vi "UHR-Fleezers Control (host) - Avogadro v1.vi"() -> ()   [LabVIEW 2014] (continued)
            n459 = local write "Stage Moving"(TRUE ("Stage Moving")) -> ()
            n460 = local write "Start Saving"(TRUE ("Start Saving")) -> ()
            n461 = call "Set Stage Position.vi"("Position"=w813, "error in"=w812, "VISA resource name in"=w811) -> ("error out"=w809:errorcluster, "VISA resource name out"=w810:refnum<visa-resource-name>)  [unwired: 1 out]
          }
          frame #2 {
            # "go back to start"
            n462 = call "Set Stage Position.vi"("Position"=w815, "error in"=w816, "VISA resource name in"=w817) -> ()  [unwired: 3 out]
          }
          frame #3 {
            # "stop saving"
            n463 = local write "Stop Saving"(TRUE ("Stop Saving")) -> ()
            n464 = local write "Stage Moving"(FALSE ("Stage Moving")) -> ()
          }
        }
      }
      event "Move to Position 1", "Move to Position 2", "Move to Position 3", "Move to Position 4", "Move to Position 5", "Lower Ch. Cap.", "Move to Position 6": Value Change {
        w820 = FALSE
        n465 = event-data() -> ()  [unwired: 1 in, 5 out]
        n466 = Or(x="Move to Position 5", y="Lower Ch. Cap.") -> (x .or. y?=w825:bool)
        n467 = Build Array("Move to Position 1", "Move to Position 2", "Move to Position 3", "Move to Position 4", w825, "Move to Position 6") -> (w828:bool[])
        n468 = local write "Move to Position 1"(w820) -> ()
        n469 = local write "Move to Position 2"(w820) -> ()
        n470 = local write "Move to Position 3"(w820) -> ()
        n471 = local write "Move to Position 4"(w820) -> ()
        n472 = local write "Move to Position 5"(w820) -> ()
        n473 = local write "Move to Position 6"(w820) -> ()
        n474 = Boolean Array To Number(Boolean array=w828) -> (number=w827:u32)
        n475 = Logarithm Base 2(1:w827) -> (0:w826:dbl)
        n476 = flat-sequence {
          tunnel: w826 -> [w837]
          tunnel: w823 -> [w835]
          tunnel: w822 -> [w834]
          frame #0 {
            n477 = local read "Saved Stage Positions"() -> (w845:dbl[][])
            n478 = Array Subset(array=w845, index (row)=w837, length (row)=1 ("length"), index (col)=1 ("index"), length (col)=3 ("length")) -> (w842:dbl[][])
            n479 = Reshape Array(w842, 3 ("dimension size")) -> (w840:dbl[])
            n480 = Array To Cluster(array=w840) -> (cluster=w839:cluster{"[0]":dbl, "[1]":dbl, "[2]":dbl})
            n481 = call "Set Stage Position.vi"("Position"=w839, "error in"=w834, "VISA resource name in"=w835) -> ("error out"=w838:errorcluster)  [unwired: 2 out]
            n482 = local write "Stage Moving"(TRUE ("Stage Moving")) -> ()
            n483 = local write "Stage Control Serial Error"(w838) -> ()
          }
          frame #1 {
            n484 = local write "Stage Moving"(FALSE ("Stage Moving")) -> ()
            n485 = call <vilib>:"Beep.vi"() -> ()  [unwired: 3 in, 9 out]
          }
        }
      }
      event "Force FB Data\nScript": Value Change {
        n486 = event-data() -> ()  [unwired: 1 in, 5 out]
        n487 = flat-sequence {
          tunnel: w853 -> [w857]
          tunnel: w854 -> [w858]
          tunnel: [w858] -> w849
          tunnel: [w857] -> w848
          tunnel: w849 -> [w861]
          tunnel: w848 -> [w860]
          tunnel: ["Trap Trig Fl."] -> w850
          tunnel: [w886] -> w851
          tunnel: w850 -> [w886]
          tunnel: [w890] -> w852
          tunnel: w851 -> [w890]
          tunnel: w852 -> [w892]
          frame #0 {
            n488 = property on="Trap Delta (MHz)" class="DigNum (strict)"("Val(Sgnl)"="Trap Delta Before Moving") -> ()  [unwired: 2 in, 2 out]
          }
          frame #1 {
            n489 = local read "Saved Stage Positions"() -> (w863:dbl[][])
            n490 = property on="Trap Pos. FB Offset Factor" class="DigNum (strict)"("Val(Sgnl)"=i64 0 ("Value (Signaling)")) -> ()  [unwired: 2 in, 2 out]
            n491 = local write "FB Trap Pos Offset"(0.0 ("FB Trap Pos Offset")) -> ()
            n492 = local write "Stage Moving"(TRUE ("Stage Moving")) -> ()
            n493 = call "move to saved stage position.vi"("error in"=w860, "Stage VISA resource name in"=w861, "Position"="Stage Position To Establish FB", "Saved Stage Positions"=w863) -> ("error out"=w859:errorcluster)  [unwired: 1 out]
            n494 = local write "Stage Control Serial Error"(w859) -> ()
          }
          frame #2 {
            n495 = call <vilib>:"Beep.vi"() -> ()  [unwired: 3 in, 9 out]
            n496 = Multiply(x="Wait (s)", y=u32 1000 ("milliseconds to wait")) -> (x*y=w870:u32)
            n497 = property on="Trap Delta (MHz)" class="DigNum (strict)"("Val(Sgnl)"="Starting \nTrap Delta (MHz)") -> ()  [unwired: 2 in, 2 out]
            n498 = local write "Stage Moving"(FALSE ("Stage Moving")) -> ()
            n499 = Wait (ms)(milliseconds to wait=w870) -> ()  [unwired: 1 out]
            n500 = property on="Tab Control 2" class="TabCtl (strict)"("Val(Sgnl)"=T11."Feedback on Trap Position" ("Value (Signaling)")) -> ()  [unwired: 2 in, 2 out]
            n501 = property on="Tab Control" class="TabCtl (strict)"("Val(Sgnl)"=T40."Trap Control (RF)" ("Value (Signaling)")) -> ()  [unwired: 2 in, 2 out]
          }
          frame #3 {
            n502 = property on="Set Reading to\nSetpoint" class="Bool (strict)"("Val(Sgnl)"=TRUE ("Value (Signaling)")) -> ()  [unwired: 2 in, 2 out]
            n503 = Wait (ms)(milliseconds to wait=u32 500) -> ()  [unwired: 1 out]
          }
          frame #4 {
            n504 = property on="Trap Pos. FB ON" class="Bool (strict)"("Val(Sgnl)"=TRUE ("Value (Signaling)")) -> ()  [unwired: 2 in, 2 out]
            n505 = Wait (ms)(milliseconds to wait=u32 250) -> ()  [unwired: 1 out]
          }
          frame #5 {
            n506 = case shown="False" "Trap Trig Fl." {
              frame False {
                n507 = case shown="True" "Green ON after FB ON?" {
                  selector: "Green ON after FB ON?" -> [_ w885]
                  frame False {
                  }
                  frame True {
                    n508 = property on="Green Laser ON" class="Bool (strict)"("Val(Sgnl)"=w885) -> ()  [unwired: 2 in, 2 out]
                  }
                }
              }
              frame True {
              }
            }
            n509 = case shown="True" "Remove Action Offset" {
              tunnel: TRUE ("Value (Signaling)") -> [w882 w883]
              frame False {
                n510 = property on="Remove Unwinding Offset" class="Bool (strict)"("Val(Sgnl)"=w882) -> ()  [unwired: 2 in, 2 out]
              }
              frame True {
                n511 = property on="Remove Action Offset" class="Bool (strict)"("Val(Sgnl)"=w883) -> ()  [unwired: 2 in, 2 out]
              }
            }
            n512 = Wait (ms)(milliseconds to wait=u32 250) -> ()  [unwired: 1 out]
          }
          frame #6 {
            n513 = property on="Start Saving" class="Bool (strict)"("Val(Sgnl)"=TRUE ("Value (Signaling)")) -> ()  [unwired: 2 in, 2 out]
            n514 = Wait (ms)(milliseconds to wait=u32 5000) -> ()  [unwired: 1 out]
          }
          frame #7 {
            w889 = TRUE ("Value (Signaling)")
            n515 = property on="Rem fb disp offset" class="Bool (strict)"("Val(Sgnl)"=w889) -> ()  [unwired: 2 in, 2 out]
            n516 = property on="Remove Offset" class="Bool (strict)"("Val(Sgnl)"=w889) -> ()  [unwired: 2 in, 2 out]
            n517 = Wait (ms)(milliseconds to wait=u32 100) -> ()  [unwired: 1 out]
          }
          frame #8 {
            n518 = case shown="True" w892 {
              frame False {
              }
              frame True {
                n519 = local write "Trap Trig. Fl."(TRUE ("Value (Signaling)")) -> ()
              }
            }
          }
          frame #9 {
            n520 = case shown="True" "Start dipping after?" {
              frame False {
              }
              frame True {
                n521 = flat-sequence {
                  frame #0 {
                    n522 = Multiply(x="Delay before dipping (s)", y=1000.0) -> (x*y=w896:dbl)
                    n523 = Wait (ms)(milliseconds to wait=w896) -> ()  [unwired: 1 out]
                  }
                  frame #1 {
                    n524 = property on="Dip for Protein" class="Bool (strict)"("Val(Sgnl)"=TRUE ("Value (Signaling)")) -> ()  [unwired: 2 in, 2 out]
                    n525 = local write "Scripts"(T2."Dipping" ("Scripts")) -> ()
                  }
                }
              }
            }
          }
        }
      }
      event "Fixed Traps Data\nScript": Value Change {
        n526 = event-data() -> ()  [unwired: 1 in, 5 out]
        n527 = flat-sequence {
          frame #0 {
            n528 = case shown="True" "Green ON" {
              frame False {
              }
              frame True {
                n529 = property on="Green Laser ON" class="Bool (strict)"("Val(Sgnl)"=TRUE) -> ()  [unwired: 2 in, 2 out]
              }
            }
            n530 = local write "Offset (nm)"(0.0 ("Offset (nm)")) -> ()
            n531 = property on="Sample Channel\nFlow" class="Bool (strict)"("Val(Sgnl)"=FALSE ("Value (Signaling)")) -> ()  [unwired: 2 in, 2 out]
            n532 = property on="Trap Delta (MHz)" class="DigNum (strict)"("Val(Sgnl)"="Fixed Traps Trap Delta (MHz)") -> ()  [unwired: 2 in, 2 out]
          }
          frame #1 {
            n533 = Wait (ms)(milliseconds to wait=u32 1000) -> ()  [unwired: 1 out]
          }
          frame #2 {
            n534 = local write "Start Saving"(TRUE ("Start Saving")) -> ()
          }
          frame #3 {
            n535 = local read "Bead Sep. Int. Time (s)"() -> (w907:dbl)
            n536 = Multiply(x=w907, y=1000.0) -> (x*y=w909:dbl)
            n537 = Wait (ms)(milliseconds to wait=w909) -> ()  [unwired: 1 out]
          }
          frame #4 {
            n538 = property on="Remove Offset" class="Bool (strict)"("Val(Sgnl)"=TRUE ("Value (Signaling)")) -> ()  [unwired: 2 in, 2 out]
          }
          frame #5 {
            n539 = property on="Dip for Protein" class="Bool (strict)"("Val(Sgnl)"="Start dipping after?") -> ()  [unwired: 2 in, 2 out]
          }
        }
      }
      event "Experiment position", "Get Bead 1", "Get bead 2", "Get bead 3": Value Change {
        w912 = FALSE
        n540 = event-data() -> ()  [unwired: 1 in, 6 out]
        n541 = Build Array("Get Bead 1", "Get bead 2", "Get bead 3", "Experiment position") -> (w917:bool[])
        n542 = Boolean Array To Number(Boolean array=w917) -> (number=w916:u32)
        n543 = local write "Get bead 3"(w912) -> ()
        n544 = local write "Get Bead 1"(w912) -> ()
        n545 = local write "Experiment position"(w912) -> ()
        n546 = local write "Get bead 2"(w912) -> ()
        n547 = Logarithm Base 2(1:w916) -> (0:w915:dbl)
        n548 = To Unsigned Long Integer(number=w915) -> (unsigned 32bit integer=w914:u32)
        n549 = case shown="3" w914 {
          frame 0, Default {
            n550 = property on="Move to Position 1" class="Bool (strict)"("Val(Sgnl)"=TRUE) -> ()  [unwired: 2 in, 2 out]
          }
          frame 1 {
            n551 = property on="Move to Position 2" class="Bool (strict)"("Val(Sgnl)"=TRUE) -> ()  [unwired: 2 in, 2 out]
          }
          frame 2 {
            n552 = property on="Move to Position 3" class="Bool (strict)"("Val(Sgnl)"=TRUE) -> ()  [unwired: 2 in, 2 out]
          }
          frame 3 {
            n553 = property on="Move to Position 4" class="Bool (strict)"("Val(Sgnl)"=TRUE) -> ()  [unwired: 2 in, 2 out]
          }
        }
      }
      event "Take Stepping Data": Value Change {
        n554 = event-data() -> ()  [unwired: 1 in, 5 out]
        n555 = local read "Save ave N"() -> (w933:dbl)
        n556 = flat-sequence {
          tunnel: w933 -> [w935]
          tunnel: [w935] -> w928
          tunnel: [w937] -> w929
          tunnel: w928 -> [w937]
          tunnel: [w939] -> w930
          tunnel: w929 -> [w939]
          tunnel: [w942] -> w931
          tunnel: w930 -> [w942]
          tunnel: [w944] -> w932
          tunnel: w931 -> [w944]
          tunnel: [w946] -> w926
          tunnel: w932 -> [w946]
          tunnel: w926 -> [w949]
          tunnel: [w949] -> w925
          tunnel: w925 -> [w950]
          tunnel: [w950] -> w927
          tunnel: w927 -> [w956]
          frame #0 {
            n557 = property on="Save ave N" class="DigNum (strict)"("Val(Sgnl)"="Save ave factor") -> ()  [unwired: 2 in, 2 out]
          }
          frame #1 {
            n558 = Wait (ms)(milliseconds to wait=u32 100) -> ()  [unwired: 1 out]
          }
          frame #2 {
            n559 = local read "Offset 2 Start (MHz)"() -> (w941:dbl)
            n560 = property on="Saved AOD Raster Scan Parameter Sets" class="Arr (strict)"("Index Values"=u32[] [2]) -> ()  [unwired: 2 in, 2 out]
            n561 = property on="Trap Delta (MHz)" class="DigNum (strict)"("Val(Sgnl)"=w941) -> ()  [unwired: 2 in, 2 out]
          }
          frame #3 {
            n562 = property on="Load parameters" class="Bool (strict)"("Val(Sgnl)"=TRUE ("Value (Signaling)")) -> ()  [unwired: 2 in, 2 out]
          }
          frame #4 {
            n563 = Wait (ms)(milliseconds to wait=u32 100) -> ()  [unwired: 1 out]
          }
          frame #5 {
            n564 = property on="Trap Raster Scan" class="Bool (strict)"("Val(Sgnl)"=TRUE ("Value (Signaling)")) -> ()  [unwired: 2 in, 2 out]
          }
          frame #6 {
            n565 = Wait (ms)(milliseconds to wait=u32 1000) -> ()  [unwired: 1 out]
          }
          frame #7 {
            n566 = while {
              stop <- w953 stop-if-true
              n567 = local read "Raster Scanning..."() -> (w955:bool)
              n568 = local read "Saving..."() -> (w954:bool)
              n569 = Not(x=w954) -> (.not. x?=w951:bool)
              n570 = Not(x=w955) -> (.not. x?=w952:bool)
              n571 = And(x=w952, y=w951) -> (x .and. y?=w953:bool)
            }
          }
          frame #8 {
            n572 = property on="Save ave N" class="DigNum (strict)"("Val(Sgnl)"=w956) -> ()  [unwired: 2 in, 2 out]
          }
        }
      }
      event "Step Size (nm)": Value Change {
        n573 = event-data() -> ()  [unwired: 1 in, 5 out]
        n574 = flat-sequence {
          frame #0 {
            n575 = property on="Saved AOD Raster Scan Parameter Sets" class="Arr (strict)"("Index Values"=u32[] [1]) -> ()  [unwired: 2 in, 2 out]
          }
          frame #1 {
            n576 = Multiply(x="N Steps", y="Step Size (nm)") -> (x*y=w958:dbl)
            n577 = property on="Scan Speed AOD (nm/s) 2" class="DigNum (strict)"("Value"="Step Size (nm)") -> ()  [unwired: 2 in, 2 out]
            n578 = property on="Step Size AOD (nm) 2" class="DigNum (strict)"("Value"="Step Size (nm)") -> ()  [unwired: 2 in, 2 out]
            n579 = property on="Scan Range AOD (nm) 2" class="DigNum (strict)"("Value"=w958) -> ()  [unwired: 2 in, 2 out]
          }
        }
      }
      event "Take Detection Laser\nImage": Value Change {
        n580 = event-data() -> ()  [unwired: 1 in, 5 out]
        n581 = flat-sequence {
          tunnel: [w986] -> w976
          tunnel: [w985] -> w969
          tunnel: [w984] -> w961
          tunnel: [w989] -> w977
          tunnel: w976 -> [w989]
          tunnel: [w988] -> w970
          tunnel: w969 -> [w988]
          tunnel: [w987] -> w962
          tunnel: w961 -> [w987]
          tunnel: [w993] -> w978
          tunnel: w977 -> [w993]
          tunnel: [w992] -> w971
          tunnel: w970 -> [w992]
          tunnel: [w991] -> w963
          tunnel: w962 -> [w991]
          tunnel: [w999] -> w979
          tunnel: w978 -> [w999]
          tunnel: [w998] -> w972
          tunnel: w971 -> [w998]
          tunnel: [w997] -> w964
          tunnel: w963 -> [w997]
          tunnel: [w1003] -> w980
          tunnel: w979 -> [w1003]
          tunnel: [w1002] -> w973
          tunnel: w972 -> [w1002]
          tunnel: [w1001] -> w965
          tunnel: w964 -> [w1001]
          tunnel: [w1007] -> w981
          tunnel: w980 -> [w1007]
          tunnel: [w1006] -> w974
          tunnel: w973 -> [w1006]
          tunnel: [w1005] -> w966
          tunnel: w965 -> [w1005]
          tunnel: [w1011] -> w982
          tunnel: w981 -> [w1011]
          tunnel: [w1010] -> w975
          tunnel: w974 -> [w1010]
          tunnel: [w1009] -> w967
          tunnel: w966 -> [w1009]
          tunnel: w982 -> [w1017]
          tunnel: w975 -> [w1016]
          tunnel: [w1014] -> w968
          tunnel: w967 -> [w1014]
          tunnel: w968 -> [w1018]
          frame #0 {
            n582 = local read "Laser interlacing mode"() -> (w985:enum32{"Laser ON", "Laser OFF", "Interlace"})
            n583 = local read "Green FB On/Off"() -> (w984:bool)
            n584 = local read "Green Laser ON"() -> (w986:bool)
          }
          frame #1 {
            n585 = property on="Green FB On/Off" class="Bool (strict)"("Val(Sgnl)"=FALSE ("Value (Signaling)")) -> ()  [unwired: 2 in, 2 out]
          }
          frame #2 {
            n586 = property on="Green Laser ON" class="Bool (strict)"("Val(Sgnl)"=TRUE ("Value (Signaling)")) -> ()  [unwired: 2 in, 2 out]
            n587 = property on="Flip Green Filter" class="Bool (strict)"("Val(Sgnl)"=TRUE ("Value (Signaling)")) -> ()  [unwired: 2 in, 2 out]
            n588 = property on="Laser interlacing mode" class="RadioBtnsControl (strict)"("Val(Sgnl)"=enum32{"Laser ON", "Laser OFF", "Interlace"}."Laser ON" ("Value (Signaling)")) -> ()  [unwired: 2 in, 2 out]
          }
          frame #3 {
            n589 = Wait (ms)(milliseconds to wait=u32 500) -> ()  [unwired: 1 out]
          }
          frame #4 {
            n590 = property on="Confocal Image" class="Bool (strict)"("Val(Sgnl)"=TRUE ("Value (Signaling)")) -> ()  [unwired: 2 in, 2 out]
          }
          frame #5 {
            n591 = Wait (ms)(milliseconds to wait=u32 2000) -> ()  [unwired: 1 out]
          }
          frame #6 {
            n592 = while {
              stop <- w1012 stop-if-true
              n593 = local read "Saving..."() -> (w1013:bool)
              n594 = Not(x=w1013) -> (.not. x?=w1012:bool)
            }
          }
          frame #7 {
            n595 = property on="Flip Green Filter" class="Bool (strict)"("Val(Sgnl)"=TRUE ("Value (Signaling)")) -> ()  [unwired: 2 in, 2 out]
            n596 = property on="Green Laser ON" class="Bool (strict)"("Val(Sgnl)"=w1017) -> ()  [unwired: 2 in, 2 out]
            n597 = property on="Laser interlacing mode" class="RadioBtnsControl (strict)"("Val(Sgnl)"=w1016) -> ()  [unwired: 2 in, 2 out]
          }
          frame #8 {
            n598 = property on="Green FB On/Off" class="Bool (strict)"("Val(Sgnl)"=w1018) -> ()  [unwired: 2 in, 2 out]
          }
        }
      }
      event "Move in a Circle": Value Change {
        w1020 = dbl[] []
        # "converting distance (d) to angle (a)\na=arcsin(d/2r)"
        # "radius"
        # "radius"
        # "T1 Y"
        # "T1 X"
        n599 = event-data() -> ()  [unwired: 1 in, 5 out]
        n600 = local read "BD 1 Frequency 1 (MHz)"() -> (w1028:dbl)
        n601 = local read "BD 2 Frequency 1 (MHz)"() -> (w1027:dbl)
        n602 = local read "BD 1 Frequency 2 (MHz)"() -> (w1026:dbl)
        n603 = local read "BD 2 Frequency 2 (MHz)"() -> (w1025:dbl)
        n604 = Subtract(x=w1027, y="Center Y Frequency (MHz)") -> (x-y=w1032:dbl)
        n605 = Absolute Value(x=w1032) -> (abs(x)=w1023:dbl)
        n606 = flat-sequence {
          tunnel: w1023 -> [w1035]
          tunnel: [w1035] -> w1022
          frame #0 {
            n607 = local write "Radius (MHz)"(w1035) -> ()
          }
        }
        n608 = node-c288("Time step (ms)") -> (w1034:T35)  [unwired: 3 in]
        n609 = timed-loop {
          timing: w1034 -> [_]
          timing-out: [_] -> w1033
          tunnel: w1028 -> [w1126]
          tunnel: w1027 -> [_]
          tunnel: w1026 -> [w1130]
          tunnel: w1025 -> [_]
          tunnel: "Center Y Frequency (MHz)" -> [w1119]
          shift-right: [w1080] -> _
          shift-left: w1020 -> [w1087]
          shift-right: [w1078] -> _
          shift-left: w1020 -> [w1086]
          shift-right: [w1071] -> _
          shift-left: w1020 -> [w1084]
          shift-right: [w1069] -> _
          shift-left: w1020 -> [w1083]
          tunnel: "Move in a Circle" -> [_]
          tunnel: ["Back to start on finish?"] -> w1024
          tunnel: w1022 -> [_]
          tunnel: w1021 -> [w1101]
          tunnel: w1020 -> [w1082]
          shift-right: [w1053] -> _
          shift-left: 0.0 -> [w1051]
          i -> [w1060]
          stop <- w1124 stop-if-true
          w1068 = 0 ("index")
          w1089 = 1 ("dimension size")
          # "Keep phase within\n2pi so errors don't \nbuild"
          # "Accumulated\nphase"
          # "Current phase"
          # "Trap 2"
          # "Trap 1"
          # "ignore if N = 0"
          # "r"
          # "r"
          # "r"
          # "r"
          # "\"omega*t\""
          # "Trap 2"
          # "Trap separation (radians)"
          # "Trap 1"
          # "Offset (starts\n at bottom of\n the circle)"
          # "omega"
          n610 = node-c288() -> (w1137:i64)  [unwired: 1 in]
          n611 = Divide(x=w1137, y=1000) -> (x/y=w1056:dbl)
          n612 = Divide(x="2D Motion Trap Separation (MHz)", y="Radius (MHz)") -> (x/y=w1111:dbl)
          n613 = Negate(x=w1056) -> (-x=w1055:dbl)
          n614 = Divide(x="Trap 2 phase shift (deg)", y=360.0) -> (x/y=w1102:dbl)
          n615 = Inverse Sine(1:w1111) -> (0:w1047:dbl)
          n616 = Multiply(x=6.283185307179586, y=w1102) -> (x*y=w1048:dbl)
          n617 = Multiply(x=6.283185307179586, y="2D Motion Frequency (Hz)") -> (x*y=w1059:dbl)
          n618 = Select(t=w1056, s="Counterclockwise/Clockwise", f=w1055) -> (s? t:f=w1058:dbl)
          n619 = Multiply(x=w1059, y=w1058) -> (x*y=w1049:dbl)
          n620 = Select(t=w1047, s="Trap shift\nmethod", f=w1048) -> (s? t:f=w1046:dbl)
          n621 = Add(x=w1049, y=w1051) -> (x+y=w1052:dbl)
          n622 = Add(x=w1052, y=w1046) -> (x+y=w1108:dbl)
          n623 = Add(x=w1052, y=1.5707963267948966) -> (x+y=w1057:dbl)
          n624 = Add(x=w1108, y=1.5707963267948966) -> (x+y=w1121:dbl)
          n625 = Cosine(x=w1057) -> (cos(x)=w1135:dbl)
          n626 = Sine(x=w1057) -> (sin(x)=w1134:dbl)
          n627 = Multiply(x=w1135, y="Radius (MHz)") -> (x*y=w1128:dbl)
          n628 = Cosine(x=w1121) -> (cos(x)=w1133:dbl)
          n629 = Sine(x=w1121) -> (sin(x)=w1132:dbl)
          n630 = Multiply(x=w1134, y="Radius (MHz)") -> (x*y=w1127:dbl)
          n631 = Multiply(x=w1133, y="Radius (MHz)") -> (x*y=w1131:dbl)
          n632 = Multiply(x=w1132, y="Radius (MHz)") -> (x*y=w1129:dbl)
          n633 = Add(x=w1128, y=w1126) -> (x+y=w1077:dbl)
          n634 = Add(x=w1127, y=w1119) -> (x+y=w1075:dbl)
          n635 = Greater Or Equal?(x=w1060, y="N steps then stop") -> (x >= y?=w1118:bool)
          n636 = Add(x=w1131, y=w1130) -> (x+y=w1066:dbl)
          n637 = Add(x=w1129, y=w1119) -> (x+y=w1064:dbl)
          n638 = Not Equal To 0?(x="N steps then stop") -> (x != 0?=w1114:bool)
          n639 = And(x=w1118, y=w1114) -> (x .and. y?=w1115:bool)
          n640 = local read "Trap 1 sum mean"() -> (w1098:dbl)
          n641 = local read "Stop All"() -> (w1123:bool)
          n642 = local write "BD 1 Frequency 1 (MHz)"(w1077) -> ()
          n643 = local write "BD 2 Frequency 1 (MHz)"(w1075) -> ()
          n644 = local write "BD 1 Frequency 2 (MHz)"(w1066) -> ()
          n645 = local write "BD 2 Frequency 2 (MHz)"(w1064) -> ()
          n646 = Select(t=w1060, s="test", f=w1098) -> (s? t:f=→"Waveform Chart":dbl)
          n647 = Compound Arithmetic op=OR(w1123, "Stop Moving", w1115) -> (w1124:bool)
          n648 = local read "BD 1 Frequency 3 (MHz)"() -> (w1107:dbl)
          n649 = local read "BD 2 Frequency 3 (MHz)"() -> (w1106:dbl)
          n650 = Select(t=w1082, s="Reset graph", f=w1083) -> (s? t:f=w1063:dbl[])
          n651 = Select(t=w1082, s="Reset graph", f=w1084) -> (s? t:f=w1065:dbl[])
          n652 = Select(t=w1082, s="Reset graph", f=w1086) -> (s? t:f=w1074:dbl[])
          n653 = Select(t=w1082, s="Reset graph", f=w1087) -> (s? t:f=w1076:dbl[])
          n654 = Initialize Array(w1064, w1089) -> (w1090:dbl[])
          n655 = Initialize Array(w1075, w1089) -> (w1093:dbl[])
          n656 = Initialize Array(w1066, w1089) -> (w1091:dbl[])
          n657 = Initialize Array(w1077, w1089) -> (w1094:dbl[])
          n658 = local read "Y RF Frequency Limits (MHz)"() -> (w1104:T23)
          n659 = local read "X RF Frequency Limits (MHz)"() -> (w1105:T23)
          n660 = call "set RF board frequency - interlace.vi"("Board 2 Frequency Limits"=w1104, "Board 1 Frequency Limits"=w1105, "FPGA VI Reference In"=w1101, "Board 2 Frequency 3 (MHz)"=w1106, "Board 1 Frequency 3 (MHz)"=w1107, "Board 2 Frequency 2 (MHz)"=w1064, "Board 2 Frequency 1 (MHz)"=w1075, "Board 1 Frequency 2 (MHz)"=w1066, "Board 1 Frequency 1  (MHz)"=w1077) -> ()  [unwired: 1 in, 2 out]
          n661 = Bundle(w1091, w1090) -> (w1062:cluster{dbl[], dbl[]})  [unwired: 1 in]
          n662 = Bundle(w1094, w1093) -> (w1092:cluster{dbl[], dbl[]})  [unwired: 1 in]
          n663 = Build Array (concatenate)(w1077, w1076) -> (w1081:dbl[])
          n664 = Build Array (concatenate)(w1075, w1074) -> (w1079:dbl[])
          n665 = Build Array (concatenate)(w1066, w1065) -> (w1072:dbl[])
          n666 = Build Array (concatenate)(w1064, w1063) -> (w1070:dbl[])
          n667 = Bundle(w1081, w1079) -> (w1061:cluster{dbl[], dbl[]})  [unwired: 1 in]
          n668 = Bundle(w1072, w1070) -> (w1088:cluster{dbl[], dbl[]})  [unwired: 1 in]
          n669 = Build Array(w1092, w1062, w1061, w1088) -> (→"Trap trajectories":cluster{dbl[], dbl[]}[])
          n670 = case "To pause the process" shown="True" "Pause rotation" {
            frame False {
            }
            frame True {
              n671 = while {
                stop <- w1140 stop-if-true
                n672 = local read "Pause rotation"() -> (w1141:bool)
                n673 = Wait (ms)(milliseconds to wait=u32 10) -> ()  [unwired: 1 out]
                n674 = Not(x=w1141) -> (.not. x?=w1140:bool)
              }
            }
          }
          n675 = Decrement(x="N steps to plot") -> (x-1=w1067:i32)
          n676 = Array Subset(array=w1079, index=w1068, length=w1067) -> (w1078:dbl[])
          n677 = Array Subset(array=w1081, index=w1068, length=w1067) -> (w1080:dbl[])
          n678 = Array Subset(array=w1072, index=w1068, length=w1067) -> (w1071:dbl[])
          n679 = Array Subset(array=w1070, index=w1068, length=w1067) -> (w1069:dbl[])
          n680 = Quotient & Remainder(x=w1052, y=6.283185307179586) -> (x-y*floor(x/y)=w1053:dbl)  [unwired: 1 out]
          n681 = node-c288() -> ()  [unwired: 1 in, 1 out]
        }
        n682 = node-c288(w1033) -> ()  [unwired: 1 out]
        n683 = case shown="True" w1024 {
          tunnel: w1028 -> [_ w1039]
          tunnel: w1027 -> [_ w1038]
          tunnel: w1026 -> [_ w1037]
          tunnel: w1025 -> [_ w1036]
          frame False {
          }
          frame True {
            n684 = flat-sequence {
              tunnel: w1039 -> [w1043]
              tunnel: w1038 -> [w1042]
              tunnel: w1037 -> [w1041]
              tunnel: w1036 -> [w1040]
              frame #0 {
                n685 = local write "BD 1 Frequency 1 (MHz)"(w1043) -> ()
                n686 = local write "BD 2 Frequency 1 (MHz)"(w1042) -> ()
                n687 = local write "BD 1 Frequency 2 (MHz)"(w1041) -> ()
                n688 = local write "BD 2 Frequency 2 (MHz)"(w1040) -> ()
              }
              frame #1 {
                n689 = property on="Update all trap values" class="Bool (strict)"("Val(Sgnl)"=TRUE ("Value (Signaling)")) -> ()  [unwired: 2 in, 2 out]
              }
            }
          }
        }
      }
      event "Stop All": Value Change {
        # "Stopping blue laser before shutting off program"
        n690 = event-data() -> ()  [unwired: 1 in, 5 out]
        n691 = local read "Delay (ms)"() -> (w1151:i32)
        n692 = call "serial write macro.vi"("String"="l0", "Delay (ms)"=w1151, "VISA resource name"=w1154) -> ("read buffer"=w1149:string, "error out"=w1150:errorcluster, "VISA resource name out"=w1153:refnum<visa-resource-name>)
        n693 = local write "read blue buffer"(w1149) -> ()
        n694 = local write "Blue Error Out"(w1150) -> ()
        n695 = VISA Close(VISA resource name=w1153) -> ()  [unwired: 1 in, 1 out]
        n696 = local read "Stop All"() -> (w1155:bool)
      }
      event "Sensitivity", "Offset Current Sign", "Offset Current Value", "Offset Current", "Bias Voltage", "Bias Voltage (mV)", "Filter Type", "Lowpass 3dB Point", "Highpass 3dB Point", "Filter Reset", "Invert Signal", "Gain Mode", "Send Command": Value Change {
        w1162 = 250 ("Delay (ms)")
        n697 = event-data() -> ()  [unwired: 1 in, 5 out]
        n698 = event shown="[0] \"Sensitivity\": Value Change" {
          selector: _ -> [_ _ _ _ _ _ _ _ _ _ _ _ _]
          dyn-events: _ -> [_ _ _ _ _ _ _ _ _ _ _ _ _]
          timeout: _ -> [_ _ _ _ _ _ _ _ _ _ _ _ _]
          tunnel: [w1174 w1182 w1190 w1199 w1209 w1217 w1220 w1224 w1227 w1230 w1233 w1240 "Command"] -> w1161
          tunnel: [w1169 w1176 w1186 w1193 w1203 w1213 _ _ _ _ _ w1236 _] -> w1156
          event "Sensitivity": Value Change {
            n699 = event-data() -> ()  [unwired: 1 in, 5 out]
            n700 = property on="Sensitivity" class="CmbBox"() -> ("Value"=→"Gain":string)  [unwired: 2 in, 2 out]
            n701 = Concatenate Strings("SENS ", "Sensitivity") -> (w1174:string)
            n702 = local read "Gain"() -> (w1171:string)
            n703 = Concatenate Strings("gain set at ", w1171) -> (w1169:string)
          }
          event "Offset Current Sign": Value Change {
            n704 = event-data() -> ()  [unwired: 1 in, 4 out]
            n705 = Boolean To (0,1)(Boolean="Offset Current Sign") -> (0, 1=w1185:i16)
            n706 = Select(t="positive", s="Offset Current Sign", f="negative") -> (s? t:f=w1177:string)
            n707 = Number To Decimal String(number=w1185) -> (decimal integer string=w1184:string)  [unwired: 1 in]
            n708 = Concatenate Strings("IOSN " ("string"), w1184) -> (w1182:string)
            n709 = Concatenate Strings("offset current sign ", w1177) -> (w1176:string)
          }
          event "Offset Current Value": Value Change {
            n710 = event-data() -> ()  [unwired: 1 in, 5 out]
            n711 = property on="Offset Current Value" class="CmbBox"() -> ("Value"=→"Read offset current":string)  [unwired: 2 in, 2 out]
            n712 = local read "Read offset current"() -> (w1187:string)
            n713 = Concatenate Strings("IOLV ", "Offset Current Value") -> (w1190:string)
            n714 = Concatenate Strings("offset current value ", w1187) -> (w1186:string)
          }
          event "Offset Current": Value Change {
            n715 = event-data() -> ()  [unwired: 1 in, 5 out]
            n716 = Boolean To (0,1)(Boolean="Offset Current") -> (0, 1=w1202:i16)
            n717 = Select(t="on", s="Offset Current", f="off") -> (s? t:f=w1194:string)
            n718 = Number To Decimal String(number=w1202) -> (decimal integer string=w1201:string)  [unwired: 1 in]
            n719 = Concatenate Strings("IOON " ("string"), w1201) -> (w1199:string)
            n720 = Concatenate Strings("offset current ", w1194) -> (w1193:string)
          }
          event "Bias Voltage": Value Change {
            n721 = event-data() -> ()  [unwired: 1 in, 5 out]
            n722 = Boolean To (0,1)(Boolean="Bias Voltage") -> (0, 1=w1210:i16)
            n723 = Number To Decimal String(number=w1210) -> (decimal integer string=w1211:string)  [unwired: 1 in]
            n724 = Select(t="on", s="Bias Voltage", f="off") -> (s? t:f=w1204:string)
            n725 = Concatenate Strings("BSON " ("string"), w1211) -> (w1209:string)
            n726 = Concatenate Strings("bias voltage", w1204) -> (w1203:string)
          }
          event "Bias Voltage (mV)": Value Change {
            n727 = event-data() -> ()  [unwired: 1 in, 5 out]
            n728 = Number To Decimal String(number="Bias Voltage (mV)") -> (decimal integer string=w1219:string)  [unwired: 1 in]
            n729 = Number To Fractional String(number="Bias Voltage (mV)") -> (F-format string=w1214:string)  [unwired: 3 in]
            n730 = Concatenate Strings("BSLV " ("string"), w1219) -> (w1217:string)
            n731 = Concatenate Strings("bias voltage value ", w1214) -> (w1213:string)
          }
          event "Filter Type": Value Change {
            n732 = event-data() -> ()  [unwired: 1 in, 5 out]
            n733 = Concatenate Strings("FLTT " ("string"), "Filter Type") -> (w1220:string)
          }
          event "Lowpass 3dB Point": Value Change {
            n734 = event-data() -> ()  [unwired: 1 in, 5 out]
            n735 = Concatenate Strings("LFRQ " ("string"), "Lowpass 3dB Point") -> (w1224:string)
          }
          event "Highpass 3dB Point": Value Change {
            n736 = event-data() -> ()  [unwired: 1 in, 5 out]
            n737 = Concatenate Strings("HFRQ " ("string"), "Highpass 3dB Point") -> (w1227:string)
          }
          event "Filter Reset": Value Change {
            n738 = event-data() -> ()  [unwired: 1 in, 5 out]
            n739 = Select(t="ROLD", s="Filter Reset", f="") -> (s? t:f=w1230:string)
          }
          event "Gain Mode": Value Change {
            n740 = event-data() -> ()  [unwired: 1 in, 5 out]
            n741 = Concatenate Strings("GNMD " ("string"), "Gain Mode") -> (w1233:string)
          }
          event "Invert Signal": Value Change {
            n742 = event-data() -> ()  [unwired: 1 in, 5 out]
            n743 = Boolean To (0,1)(Boolean="Invert Signal") -> (0, 1=w1243:i16)
            n744 = Number To Decimal String(number=w1243) -> (decimal integer string=w1242:string)  [unwired: 1 in]
            n745 = Concatenate Strings("INVT " ("string"), w1242) -> (w1240:string)
            n746 = Select(t="signal inverted", s="Invert Signal", f="signal not inverted") -> (s? t:f=w1236:string)
          }
          event "Send Command": Value Change {
            n747 = event-data() -> ()  [unwired: 1 in, 5 out]
          }
        }
        "Command Sent" <- w1161
        n748 = local read "Save Event Log?"() -> (w1157:bool)
        n749 = local read "Saving..."() -> (w1158:bool)
        n750 = And(x=w1157, y=w1158) -> (x .and. y?=w1159:bool)
        n751 = case shown="True" w1159 {
          tunnel: w1156 -> [_ w1166]
          frame False {
          }
          frame True {
            n752 = local read "Time (s)"() -> (w1167:dbl)
            n753 = local read "log file ref"() -> (w1168:refnum<file>)
            n754 = call "write to event log.vi"("log file ref"=w1168, "time"=w1167, "input string"=w1166) -> ()  [unwired: 8 in]
          }
        }
        n755 = call "preamp serial write macro.vi"("String"=w1161, "Delay (ms)"=w1162, "VISA resource name"=w1165) -> ("read buffer"=→"Reply":string, "error out"=w1164:errorcluster)  [unwired: 1 out]
        n756 = call "preamp serial write macro.vi"("String"=w1161, "Delay (ms)"=w1162, "VISA resource name"=w1160) -> ()  [unwired: 3 out]
        n757 = local write "Preamp Error Out"(w1164) -> ()
      }
    }
    n758 = node-c288() -> ()  [unwired: 1 in, 1 out]
  }
  n759 = xnode "Open FPGA VI Reference"("resource name"=T27 "RIO0") -> ("FPGA VI Reference Out"=w30:T41, "error out"=w29:errorcluster)  [unwired: 1 in]
  n760 = xnode "Invoke Method"("FPGA VI Reference In"=w30, "error in"=w29) -> ("FPGA VI Reference Out"=w11:T41, "error out"=→"FPGA error out":errorcluster)
  n761 = Subtract(x=w9, y="Maximum Delta\n(MHz)") -> (x-y=w7:dbl)
  n762 = Bundle By Name(cluster=T23 {"Minimum"=60.0, "Maximum"=90.0, "Increment"=1.0} ("Min Max Inc"), "Minimum"=w7, "Maximum"=w9) -> (w6:T23)
  n763 = flat-sequence "Safety limits on RF frequencies and amplitudes (for AOM protection)" {
    tunnel: [w1247] -> w21
    tunnel: [w1245] -> w23
    tunnel: [w1248] -> w24
    tunnel: [w1249] -> w22
    tunnel: w6 -> [w1247]
    tunnel: T23 {"Minimum"=0.0, "Maximum"=50.0, "Increment"=1.0} ("Data Entry Limits") -> [w1245]
    tunnel: w11 -> [w1246]
    tunnel: [w1246] -> w25
    frame #0 {
      w1249 = T23 {"Minimum"=0.0, "Maximum"=40.0, "Increment"=0.1} ("Min Max Inc")
      w1248 = T23 {"Minimum"=0.0, "Maximum"=45.0, "Increment"=1.0} ("Data Entry Limits")
      n764 = property on="BD 2 Frequency 1 (MHz)" class="DigNum (strict)"("Data Range"=w1249) -> ()  [unwired: 2 in, 2 out]
      n765 = property on="BD 2 Frequency 3 (MHz)" class="DigNum (strict)"("Data Range"=w1249) -> ()  [unwired: 2 in, 2 out]
      n766 = property on="BD 2 Frequency 2 (MHz)" class="DigNum (strict)"("Data Range"=w1249) -> ()  [unwired: 2 in, 2 out]
      n767 = property on="BD 1 Frequency 1 (MHz)" class="DigNum (strict)"("Data Range"=w1247) -> ()  [unwired: 2 in, 2 out]
      n768 = property on="BD 1 Frequency 2 (MHz)" class="DigNum (strict)"("Data Range"=w1247) -> ()  [unwired: 2 in, 2 out]
      n769 = property on="BD 1 Frequency 3 (MHz)" class="DigNum (strict)"("Data Range"=w1247) -> ()  [unwired: 2 in, 2 out]
      n770 = property on="BD 2 Amplitude 1 (%)" class="DigNum (strict)"("Data Range"=w1248) -> ()  [unwired: 2 in, 2 out]
      n771 = property on="BD 2 Amplitude 2 (%)" class="DigNum (strict)"("Data Range"=w1248) -> ()  [unwired: 2 in, 2 out]
      n772 = property on="BD 2 Amplitude 3 (%)" class="DigNum (strict)"("Data Range"=w1248) -> ()  [unwired: 2 in, 2 out]
      n773 = property on="BD 1 Amplitude 3 (%)" class="DigNum (strict)"("Data Range"=w1245) -> ()  [unwired: 2 in, 2 out]
      n774 = property on="BD 1 Amplitude 2 (%)" class="DigNum (strict)"("Data Range"=w1245) -> ()  [unwired: 2 in, 2 out]
      n775 = property on="BD 1 Amplitude 1 (%)" class="DigNum (strict)"("Data Range"=w1245) -> ()  [unwired: 2 in, 2 out]
      "X RF Frequency Limits (MHz)" <- w1247
      "X RF Amplitude Limits (%)" <- w1245
      "Y RF Amplitude Limits (%)" <- w1248
      "Y RF Frequency Limits (MHz)" <- w1249
    }
  }
  n776 = stacked-sequence "Host initialization sequence - order matters!" {
    tunnel: w25 -> [_ w1269 w1361 _ w1418 w1427 w1494 w1518 _ w1588]
    tunnel: [_ _ _ _ _ _ _ _ _ w1588] -> w14
    tunnel: [_ _ _ _ _ _ _ _ _ w1587] -> w27
    tunnel: w24 -> [_ _ _ _ _ _ w1492 _ _ _]
    tunnel: w23 -> [_ _ _ _ _ _ w1491 _ _ _]
    tunnel: w22 -> [_ _ _ _ _ _ w1490 _ _ _]
    tunnel: w21 -> [_ _ _ _ _ _ w1471 _ _ _]
    tunnel: [_ _ _ _ _ _ _ _ w1585 _] -> _
    tunnel: w1 -> [_ _ _ _ _ _ _ _ w1547 _]
    frame #0 {
    }
    frame #1 {
      w1301 = 10.0 ("y")
      w1302 = 32767.0 ("y")
      w1286 = 6.0  # clock mult.
      w1285 = 49152000.0  # TCXO frequ.
      # "Initialize some FPGA settings"
      n777 = local read "Not-Interlacing Set"() -> (w1341:enum32{"Set 1", "Set 2", "Set 3"})
      n778 = local write "Trap Pos FIFO Timeout"(u16 0 ("Trap Pos FIFO Timeout")) -> ()
      n779 = local read "Interlace"() -> (w1339:bool)
      n780 = local read "Desired Scan Incr (V)"() -> (w1313:dbl)
      n781 = local read "BD 1 Delay (ticks)"() -> (w1348:u8)
      n782 = local read "Number Interlace Sets"() -> (w1340:u8)
      n783 = local read "BD 2 Delay (Ticks)"() -> (w1349:u8)
      n784 = property on="AI Count (ticks)" class="DigNum (strict)"("Val(Sgnl)"="AI Count (ticks)") -> ()  [unwired: 2 in, 2 out]
      n785 = local read "AO1"() -> (w1307:dbl)
      n786 = local read "AO2"() -> (w1308:dbl)
      n787 = local read "Next trap write delay (ticks)"() -> (w1350:u8)
      n788 = local read "Number of scans (MCL)"() -> (w1317:u64)
      n789 = local read "Cycles/step (MCL)"() -> (w1316:u64)
      n790 = local read "Scan steps (MCL)"() -> (w1315:u64)
      n791 = local read "Continuous MCL Scanning"() -> (w1318:bool)
      n792 = Multiply(x=w1307, y=w1302) -> (x*y=w1305:dbl)
      n793 = Multiply(x=w1308, y=w1302) -> (x*y=w1303:dbl)
      n794 = Build Array("DIO count 1 (ticks)", "DIO count 2 (ticks)", "DIO count 3 (ticks)") -> (w1334:u16[])
      n795 = local read "Fast Scan Dir"() -> (w1319:bool)
      n796 = local read "2D or 1D Scan"() -> (w1331:bool)
      n797 = local read "N Acq Sets (Traps + Fl.)"() -> (w1327:i16)
      n798 = local read "Scan Increment (MHz)"() -> (w1290:dbl)
      n799 = Divide(x=w1305, y=w1301) -> (x/y=w1306:dbl)
      n800 = Divide(x=w1303, y=w1301) -> (x/y=w1304:dbl)
      n801 = To Unsigned Byte Integer(number=w1341) -> (unsigned 8bit integer=w1336:u8)
      n802 = Split 1D Array(array=w1334, index=w1340) -> (first subarray=w1332:u16[])  [unwired: 1 out]
      n803 = Multiply(x=w1313, y=32767.0) -> (x*y=w1311:dbl)
      n804 = To Word Integer(number=w1306) -> (16bit integer=w1252:i16)
      n805 = To Word Integer(number=w1304) -> (16bit integer=w1251:i16)
      n806 = Index Array(array=w1334, index=w1336) -> (element=w1335:u16)
      n807 = Add Array Elements(numeric array=w1332) -> (sum=w1333:u16)
      n808 = Multiply(x=w1285, y=w1286) -> (x*y=w1287:dbl)
      n809 = Divide(x=w1311, y=10.0) -> (x/y=w1312:dbl)
      n810 = Select(t=w1333, s=w1339, f=w1335) -> (s? t:f=w1342:u16)
      n811 = Not(x=w1319) -> (.not. x?=w1320:bool)
      n812 = To Word Integer(number=w1312) -> (16bit integer=w1314:i16)
      n813 = property on="2D or 1D Scan" class="Bool (strict)"("Val(Sgnl)"=w1331) -> ()  [unwired: 2 in, 2 out]
      n814 = Divide(x=40000000.0, y="AI Count (ticks)") -> (x/y=w1323:dbl)
      n815 = local write "Update Count (MCL)"(w1342) -> ()
      n816 = local write "Total Counts (ticks)"(w1342) -> ()
      n817 = Divide(x=w1323, y="FPGA Ave.") -> (x/y=w1322:dbl)
      n818 = local write "AI rate (Hz)"(w1323) -> ()
      n819 = Multiply(x=w1290, y=1000.0) -> (x*y=w1283:dbl)
      n820 = local write "Ave. Rate (Hz)"(w1322) -> ()
      n821 = Reciprocal(x=w1322) -> (1/x=w1321:dbl)
      n822 = Scale By Power Of 2(n=48, x=w1283) -> (x*2^n=w1282:dbl)
      n823 = local write "Ave. Period (s)"(w1321) -> ()
      n824 = Divide(x=w1282, y=w1287) -> (x/y=w1288:dbl)
      n825 = To Quad Integer(1:w1288) -> (0:w1291:i64)
      n826 = local read "Setpoints (V)"() -> (w1276:cluster{"Set 1":dbl, "Set 2":dbl})
      n827 = local read "# Samples/channel"() -> (w1298:u32)
      n828 = local read "Feedback On/Off"() -> (w1273:cluster{"Set 1":bool, "Set 2":bool})
      n829 = local read "T3 Y (V)"() -> (w1256:dbl)
      n830 = local read "T3 X (V)"() -> (w1255:dbl)
      n831 = local read "Trap intensity output range"() -> (w1266:cluster{"Normal High":i16, "Normal Low":i16})
      n832 = local read "All FB On/Off"() -> (w1272:bool)
      n833 = local read "Number of F/B Scans (AOD)"() -> (w1297:u16)
      n834 = local read "Trap Intensity PID Gains"() -> (w1265:T14)
      n835 = local read "Cycles/step (AOD)"() -> (w1293:u64)
      n836 = local read "Scan steps (AOD)"() -> (w1292:u64)
      n837 = Multiply(x=w1292, y=w1293) -> (x*y=w1294:u64)
      n838 = Multiply(x=w1294, y=u64 2) -> (x*y=w1296:u64)
      n839 = Multiply(x=w1296, y=w1297) -> (x*y=w1299:u64)
      n840 = Multiply(x=3276.7, y=w1276) -> (x*y=w1277:cluster{"Set 1":dbl, "Set 2":dbl})
      n841 = local read "Scan BD"() -> (w1281:bool)
      n842 = Multiply(x=w1256, y=32767.0) -> (x*y=w1262:dbl)
      n843 = And(x=w1273, y=w1272) -> (x .and. y?=w1274:cluster{"Set 1":bool, "Set 2":bool})
      n844 = To Word Integer(number=w1277) -> (16bit integer=w1278:cluster{"Set 1":i16, "Set 2":i16})
      n845 = Multiply(x=w1255, y=32767.0) -> (x*y=w1259:dbl)
      n846 = local read "Sets to FIFO (Traps)"() -> (w1344:T22)
      n847 = Divide(x=w1299, y=w1298) -> (x/y=w1300:dbl)
      n848 = Unbundle By Name(w1274) -> ("Set 1"=w1270:bool, "Set 2"=w1271:bool)
      n849 = Unbundle By Name(w1278) -> ("Set 1"=w1279:i16, "Set 2"=w1280:i16)
      n850 = Divide(x=w1262, y=10.0) -> (x/y=w1263:dbl)
      n851 = Divide(x=w1259, y=10.0) -> (x/y=w1258:dbl)
      n852 = To Unsigned Word Integer(number=w1263) -> (unsigned 16bit integer=w1254:u16)
      n853 = To Unsigned Word Integer(number=w1258) -> (unsigned 16bit integer=w1253:u16)
      n854 = local read "FPGA error out"() -> (w1268:errorcluster)
      n855 = local write "Data points/scan (f/b)"(w1296) -> ()
      n856 = local write "Data points/scans"(w1299) -> ()
      n857 = local write "N sets should be saved"(w1300) -> ()
      n858 = Unbundle By Name(w1344) -> ("Set 1"=w1345:bool, "Set 2"=w1346:bool, "Set 3"=w1347:bool)
      n859 = xnode "Read/Write Control"("FPGA VI Reference In"=w1269, "error in"=w1268, "ai count"="AI Count (ticks)", "Interlace ON/OFF"=w1339, "Number Interlace Cycles"=w1340, "Set 1"=w1345, "Set 2"=w1346, "Set 3"=w1347, "FB On/Off Set 1"=w1270, "FB On/Off Set 2"=w1271, "Interlace Off Parameters"=w1341, "FB Setpoint Set 1"=w1279, "FB Setpoint Set 2"=w1280, "Piezo Trap Y (AO4)"=w1254, "Piezo Trap X (AO5)"=w1253, "FB Gains"=w1265, "FB output range"=w1266, "Cycles per step"=w1293, "Scan BD"=w1281, "Number of scans"=w1297, "Scan steps"=w1292, "Scan freq.  increment"=w1291, "AO1 (Y)"=w1252, "AO2 (X)"=w1251, "Scan freq.  increment (MCL)"=w1314, "Scan steps (MCL)"=w1315, "Cycles per step (MCL)"=w1316, "Number of scans (MCL)"=w1317, "MCL count"=w1342, "Cont. Scan (MCL)"=w1318, "MCL Scan Axis"=w1320, "1D or 2D Scan?"=w1331, "N of AI1 Int Acq Sets"=w1327, "Amp switch delay"="Amp switch delay", "Swap F1 and F2"="Swap F1 and F2", "APD to FIFO"=FALSE, "DIO count 1 (ticks)"="DIO count 1 (ticks)", "DIO count 2 (ticks)"="DIO count 2 (ticks)", "DIO count 3 (ticks)"="DIO count 3 (ticks)", "BD 1 Delay (ticks)"=w1348, "BD 2 Delay (Ticks)"=w1349, "Next trap write delay (ticks)"=w1350) -> ("error out"=w1267:errorcluster)  [unwired: 1 out]
      n860 = local write "FPGA error out"(w1267) -> ()
    }
    frame #2 {
      # "Initialize some more FPGA settings"
      n861 = local read "Trap Pos FB Monitor\nT1 or T2"() -> (w1372:bool)
      n862 = local read "Trap Pos FB Negate Action"() -> (w1373:bool)
      n863 = local read "Trap Pos. FB Offset Factor"() -> (w1374:i64)
      n864 = local read "Trap Pos. FB Mult Factor"() -> (w1375:i64)
      n865 = local read "Trap Pos. AI1 X Pre-scale"() -> (w1377:u16)
      n866 = local read "Trap Pos FB Int Count"() -> (w1379:u16)
      n867 = local read "Green Laser ON"() -> (w1351:bool)
      n868 = local read "Neg. TTrig FPGA"() -> (w1380:bool)
      n869 = local read "Trap Pos. FB Range"() -> (w1356:T18)
      n870 = local read "Trap Pos. FB Gains"() -> (w1357:T17)
      n871 = local read "Dynamic Force FB (ronen)"() -> (w1358:bool)
      n872 = Multiply(x="Green Intensity % (FB OFF)", y=655.35) -> (x*y=w1366:dbl)
      n873 = Multiply(x="Red FB Setpoint (mV)", y=3.2767) -> (x*y=w1388:dbl)
      n874 = Multiply(x="Red Intensity % (FB OFF)", y=655.35) -> (x*y=w1392:dbl)
      n875 = Unbundle By Name("Red FB Gains") -> ("proportional gain (Kc)"=w1397:i16, "integral gain (Kc*Ts/Ti)"=w1398:i16, "derivative gain (Kc*Td/Ts)"=w1399:i16)
      n876 = Multiply(x="Green FB Setpoint (mV)", y=3.2767) -> (x*y=w1369:dbl)
      n877 = To Unsigned Word Integer(number=w1366) -> (unsigned 16bit integer=w1368:u16)
      n878 = To Unsigned Word Integer(number=w1392) -> (unsigned 16bit integer=w1395:u16)
      n879 = To Word Integer(number=w1388) -> (16bit integer=w1391:i16)
      n880 = local read "Differential FB?"() -> (w1382:bool)
      n881 = To Word Integer(number=w1369) -> (16bit integer=w1371:i16)
      n882 = local read "Laser interlacing mode"() -> (w1354:enum32{"Laser ON", "Laser OFF", "Interlace"})
      n883 = local read "Invert laser interlacing"() -> (w1355:bool)
      n884 = Unbundle By Name("Green FB Gains") -> ("proportional gain (Kc)"=w1385:i16, "integral gain (Kc*Ts/Ti)"=w1386:i16, "derivative gain (Kc*Td/Ts)"=w1387:i16)
      n885 = Select(t=w1354, s=w1351, f=enum32{"Laser ON", "Laser OFF", "Interlace"}."Laser OFF" ("Green laser mode")) -> (s? t:f=w1353:enum32{"Laser ON", "Laser OFF", "Interlace"})
      n886 = local read "FPGA error out"() -> (w1359:errorcluster)
      n887 = xnode "Read/Write Control"("FPGA VI Reference In"=w1361, "error in"=w1359, "Invert GI"=w1355, "Invert GI 2"=w1355, "Invert RI"=w1355, "Invert RI 2"=w1355, "Operating Mode"=w1353, "Operating Mode 2"=w1353, "Red Laser Operating Mode"=w1353, "RI Operating Mode 2"=w1353, "P3"=w1385, "I3"=w1386, "D3"=w1387, "Green FB Setpoint"=w1371, "Green FB On/Off"="Green FB On/Off", "Current Out"=w1368, "Green int current ON count adj"="Green int current ON count adj", "Trap Pos FB Monitor T1 or T2"=w1372, "Trap Pos FB Negate Action"=w1373, "Trap Pos. FB Offset Factor"=w1374, "Trap Pos. FB Mult Factor"=w1375, "Force feedback"=FALSE, "AI1 X Scale"=w1377, "Trap Pos to FIFO"=TRUE, "Trap Pos FB Int Count"=w1379, "TTrig Negate Pos"=w1380, "FB Trig Integrate"="FB Trig Integrate", "Diff FB Measurement?"=w1382, "Negate Diff?"="Negate Diff?", "Trap pos. FB Range"=w1356, "Trap Pos. FB Gains"=w1357, "Red FB Setpoint"=w1391, "RI Current Out"=w1395, "P4"=w1397, "I4"=w1398, "D4"=w1399, "Red FB On/Off"="Red FB On/Off", "Dynamic Force FB (Ronen)"=w1358) -> ("error out"=w1360:errorcluster)  [unwired: 1 out]
      n888 = local write "FPGA error out"(w1360) -> ()
    }
    frame #3 {
      # "Initialize more settings. Should stop using event loops to initialize."
      # "What are these?"
      n889 = local write "Offset (nm)"(0.0 ("Offset (nm)")) -> ()
      n890 = local write "Bead Mean (nm)"(0.0 ("Bead Mean (nm)")) -> ()
      n891 = stacked-sequence {
        frame #0 {
          w1403 = T43."empty" ("mode")
          # "Clear external fluorescence triggering FIFO"
          # "APD loop counts"
          # "Fluorescence loop counts (rates)"
          n892 = local read "APD Integration Time (s)"() -> (w1405:dbl)
          n893 = local read "Interlace ON count"() -> (w1406:u16)
          n894 = call "Smart Buffer (DBL) 1.vi"("mode"=w1403) -> ()  [unwired: 5 in, 6 out]
          n895 = call "Smart Buffer (DBL) 2.vi"("mode"=w1403) -> ()  [unwired: 5 in, 6 out]
          n896 = property on="APD Integration Time (s)" class="DigNum (strict)"("Val(Sgnl)"=w1405) -> ()  [unwired: 2 in, 2 out]
          n897 = property on="Interlace ON count" class="DigNum (strict)"("Val(Sgnl)"=w1406) -> ()  [unwired: 2 in, 2 out]
          "Number of APDs" <- 3.0 ("Number of APDs")
        }
        frame #1 {
          # "Number of APDs affects\nAPD DMA transfer"
          # "General settings for all lasers:"
          # "And includes all laser\nON/OFF settings"
          # "Fluorescent lasers settings:"
          # "Blue laser settings:"
          n898 = local read "Laser interlacing mode"() -> (w1408:enum32{"Laser ON", "Laser OFF", "Interlace"})
          n899 = local read "Invert laser interlacing"() -> (w1407:bool)
          n900 = local read "Blue FB On/Off"() -> (w1409:bool)
          n901 = property on="Blue FB On/Off" class="Bool (strict)"("Val(Sgnl)"=w1409) -> ()  [unwired: 2 in, 2 out]
          n902 = property on="Invert laser interlacing" class="Bool (strict)"("Val(Sgnl)"=w1407) -> ()  [unwired: 2 in, 2 out]
          n903 = property on="Laser interlacing mode" class="RadioBtnsControl (strict)"("Val(Sgnl)"=w1408) -> ()  [unwired: 2 in, 2 out]
        }
        frame #2 {
          w1410 = path "C:/Home/Bustamante Lab/Comstock-LabView-Link.udl" ("connection information")
          # "Database link changed by Ronen - not clear if it matter for the program."
          # "Initialize the database connection"
          n904 = disable-structure shown="Disabled" {
            disable-tunnel: [w1413 _] -> w1411
            disable-tunnel: w1410 -> [w1412 _]
            frame Disabled {
              n905 = call-poly <vilib>:"DB Tools Open Connection.vi"("connection information"=w1412) -> ("connection reference"=w1413:T24)  [unwired: 7 in, 1 out]
            }
            frame Enabled {
            }
          }
          "connection reference" <- w1411
          n906 = local write "connection reference"(w1411) -> ()
          n907 = local write "Database link"(w1410) -> ()
        }
        frame #3 {
          # "Load active calibration to fpga"
          n908 = local read "Base N trap periods"() -> (w1415:u32)
          n909 = local read "T1 Osc Enable"() -> (w1414:bool)
          n910 = property on="T1 Osc Enable" class="Bool (strict)"("Val(Sgnl)"=w1414) -> ()  [unwired: 2 in, 2 out]